vi "Dresden R2R Sputter 03.02.2018 IY24.vi"() -> ()   [LabVIEW 2009] (continued)
                                }
                                frame #1 {
                                }
                                }
                                }
                                frame #1 {
                                }
                                }
                                }
                                frame #5 {
                                n21432 = local read "Semi"() -> (w22479:bool)
                                n21433 = case shown="False" w22479 {
                                frame #0 {
                                n21434 = while {
                                i -> [w22485]
                                stop <- w22481 stop-if-true
                                n21435 = local read "Pc_bv_opened_ch4"() -> (w22483:bool)
                                n21436 = Greater?(x=w22485, y=120) -> (0:w22484:bool)
                                n21437 = local read "Semi"() -> (w22482:bool)
                                n21438 = Compound Arithmetic op=OR(w22482, w22483, w22484) -> (w22481:bool)
                                n21439 = Wait (ms)(milliseconds to wait=u32 500) -> ()  [unwired: 1 out]
                                }
                                }
                                frame #1 {
                                }
                                }
                                }
                                frame #6 {
                                n21440 = local read "Semi"() -> (w22487:bool)
                                n21441 = case shown="False" w22487 {
                                frame #0 {
                                n21442 = local read "Pc_bv_opened_ch4"() -> (w22488:bool)
                                n21443 = case shown="False" w22488 {
                                frame #0 {
                                n21444 = local write "Error Message"("Start up process  cancelled\nbecause  PC-BV not opened.\nPlease check PC-BV4 connections." ("Error Message")) -> ()
                                n21445 = Wait (ms)(milliseconds to wait=u32 1000) -> ()  [unwired: 1 out]
                                }
                                frame #1 {
                                }
                                }
                                }
                                frame #1 {
                                }
                                }
                                }
                                }
                                }
                                frame #1 {
                                }
                                }
                                }
                                frame #1 {
                                n21446 = local read "Semi"() -> (w22491:bool)
                                n21447 = case shown="False" w22491 {
                                frame #0 {
                                n21448 = local write "Ch4_PV13"(TRUE ("P03")) -> ()
                                n21449 = Wait Until Next ms Multiple(millisecond multiple=u32 1000) -> ()  [unwired: 1 out]
                                }
                                frame #1 {
                                }
                                }
                                }
                                }
                              }
                              frame #1 {
                              }
                            }
                          }
                          frame #9 {
                            # "OPEN/CLOSE TRNS GV-BP"
                            n21450 = local read "Semi"() -> (w22494:bool)
                            n21451 = case shown="False" w22494 {
                              frame #0 {
                                n21452 = stacked-sequence {
                                frame #0 {
                                n21453 = local read "Semi"() -> (w22495:bool)
                                n21454 = case shown="False" w22495 {
                                frame #0 {
                                n21455 = while {
                                i -> [w22504]
                                stop <- w22499 stop-if-true
                                n21456 = Greater?(x=w22504, y=50) -> (0:w22502:bool)
                                n21457 = case shown="True" w22502 {
                                frame #0 {
                                }
                                frame #1 {
                                n21458 = local read "Ch3_pressure"() -> (w22518:dbl)
                                n21459 = Less?(x=w22518, y=1) -> (x < y?=w22517:bool)
                                n21460 = case shown="True" w22517 {
                                frame #0 {
                                n21461 = local write "Error Message"("Start up process  cancelled\nbecause \n Trns GV-BP2 not closed.\nPlease check \nTrns GV-BP2 connections." ("Error Message")) -> ()
                                }
                                frame #1 {
                                n21462 = local write "Error Message"("Start up process  cancelled\nbecause\n  Trns GV-BP2 not opened.\nPlease check \nTrns GV-BP2 connections." ("Error Message")) -> ()
                                }
                                }
                                n21463 = local write "Semi"(TRUE ("Semi")) -> ()
                                }
                                }
                                n21464 = local read "Ch3_pressure"() -> (w22498:dbl)
                                n21465 = Less?(x=w22498, y=1) -> (x < y?=w22496:bool)
                                n21466 = case shown="True" w22496 {
                                tunnel: [w22506 w22512] -> w22501
                                frame #0 {
                                n21467 = local read "Ch4_Trns_gv_bp_di"() -> (w22505:bool)
                                n21468 = case shown="True" w22505 {
                                tunnel: [TRUE FALSE] -> w22506
                                frame #0 {
                                }
                                frame #1 {
                                n21469 = local write "Ch4_Trns_gv_bp_do"(FALSE ("Ch1_Tp_bv_do")) -> ()
                                n21470 = Wait Until Next ms Multiple(millisecond multiple=u32 200) -> ()  [unwired: 1 out]
                                }
                                }
                                }
                                frame #1 {
                                n21471 = local read "Ch4_Trns_gv_bp_di"() -> (w22511:bool)
                                n21472 = case shown="False" w22511 {
                                tunnel: [FALSE TRUE] -> w22512
                                frame #0 {
                                n21473 = local write "Ch4_Trns_gv_bp_do"(TRUE ("Ch1_Tp_bv_do")) -> ()
                                n21474 = Wait Until Next ms Multiple(millisecond multiple=u32 200) -> ()  [unwired: 1 out]
                                }
                                frame #1 {
                                }
                                }
                                }
                                }
                                n21475 = local read "Semi"() -> (w22500:bool)
                                n21476 = Or(x=w22501, y=w22500) -> (x .or. y?=w22499:bool)
                                }
                                }
                                frame #1 {
                                }
                                }
                                }
                                frame #1 {
                                n21477 = local read "Semi"() -> (w22523:bool)
                                n21478 = case shown="False" w22523 {
                                frame #0 {
                                n21479 = local write "Ch4_PV14"(TRUE ("P03")) -> ()
                                n21480 = Wait Until Next ms Multiple(millisecond multiple=u32 1000) -> ()  [unwired: 1 out]
                                }
                                frame #1 {
                                }
                                }
                                }
                                }
                              }
                              frame #1 {
                              }
                            }
                          }
                          frame #10 {
                            # "CHECK CH-PRESSURE"
                            n21481 = local read "Semi"() -> (w22526:bool)
                            n21482 = case shown="False" w22526 {
                              frame #0 {
                                n21483 = stacked-sequence {
                                frame #0 {
                                n21484 = local read "Semi"() -> (w22527:bool)
                                n21485 = case shown="False" w22527 {
                                frame #0 {
                                n21486 = while {
                                i -> [w22536]
                                stop <- w22531 stop-if-true
                                n21487 = Greater?(x=w22536, y=600) -> (0:w22534:bool)
                                n21488 = case shown="True" w22534 {
                                frame #0 {
                                }
                                frame #1 {
                                n21489 = local write "Semi"(TRUE ("Semi")) -> ()
                                n21490 = local write "Error Message"("Start up process was cancelled.\nPlease check chamber \nvacuum connections." ("Error Message")) -> ()
                                }
                                }
                                n21491 = local read "Ch4pressure"() -> (w22530:dbl)
                                n21492 = Less?(x=w22530, y=0.9) -> (x < y?=w22528:bool)
                                n21493 = case shown="False" w22528 {
                                tunnel: [FALSE TRUE] -> w22533
                                frame #0 {
                                n21494 = Wait Until Next ms Multiple(millisecond multiple=u32 500) -> ()  [unwired: 1 out]
                                }
                                frame #1 {
                                }
                                }
                                n21495 = local read "Semi"() -> (w22532:bool)
                                n21496 = Or(x=w22533, y=w22532) -> (x .or. y?=w22531:bool)
                                }
                                }
                                frame #1 {
                                }
                                }
                                }
                                frame #1 {
                                n21497 = local read "Semi"() -> (w22542:bool)
                                n21498 = case shown="False" w22542 {
                                frame #0 {
                                n21499 = local write "Ch4_PV15"(TRUE ("P03")) -> ()
                                n21500 = Wait Until Next ms Multiple(millisecond multiple=u32 1000) -> ()  [unwired: 1 out]
                                }
                                frame #1 {
                                }
                                }
                                }
                                }
                              }
                              frame #1 {
                              }
                            }
                          }
                          frame #11 {
                            # "OPEN BG-BV"
                            n21501 = local read "Semi"() -> (w22545:bool)
                            n21502 = case shown="False" w22545 {
                              frame #0 {
                                n21503 = stacked-sequence {
                                frame #0 {
                                n21504 = local read "Semi"() -> (w22546:bool)
                                n21505 = case shown="False" w22546 {
                                frame #0 {
                                n21506 = while {
                                i -> [w22553]
                                stop <- w22548 stop-if-true
                                n21507 = Greater?(x=w22553, y=50) -> (0:w22551:bool)
                                n21508 = case shown="True" w22551 {
                                frame #0 {
                                }
                                frame #1 {
                                n21509 = local write "Semi"(TRUE ("Semi")) -> ()
                                n21510 = local write "Error Message"("Start up process  cancelled\nbecause  BG-BV not opened.\nPlease check BG-BV4 connections." ("Error Message")) -> ()
                                }
                                }
                                n21511 = local read "Ch4_Bg_bv_di"() -> (w22547:bool)
                                n21512 = case shown="False" w22547 {
                                tunnel: [FALSE TRUE] -> w22550
                                frame #0 {
                                n21513 = Wait Until Next ms Multiple(millisecond multiple=u32 200) -> ()  [unwired: 1 out]
                                n21514 = local write "Ch4_Bg_bv_do"(TRUE ("Ch1_Tp_bv_do")) -> ()
                                }
                                frame #1 {
                                }
                                }
                                n21515 = local read "Semi"() -> (w22549:bool)
                                n21516 = Or(x=w22550, y=w22549) -> (x .or. y?=w22548:bool)
                                }
                                }
                                frame #1 {
                                }
                                }
                                }
                                frame #1 {
                                n21517 = local read "Semi"() -> (w22560:bool)
                                n21518 = case shown="False" w22560 {
                                frame #0 {
                                n21519 = local write "Ch4_PV16"(TRUE ("P03")) -> ()
                                n21520 = Wait Until Next ms Multiple(millisecond multiple=u32 1000) -> ()  [unwired: 1 out]
                                }
                                frame #1 {
                                }
                                }
                                }
                                }
                              }
                              frame #1 {
                              }
                            }
                          }
                          frame #12 {
                            # "CHECK CH-PRESSURE"
                            n21521 = local read "Semi"() -> (w22563:bool)
                            n21522 = case shown="False" w22563 {
                              frame #0 {
                                n21523 = stacked-sequence {
                                frame #0 {
                                n21524 = local read "Semi"() -> (w22564:bool)
                                n21525 = case shown="False" w22564 {
                                frame #0 {
                                n21526 = while {
                                i -> [w22573]
                                stop <- w22568 stop-if-true
                                n21527 = Greater?(x=w22573, y=240) -> (0:w22571:bool)
                                n21528 = case shown="True" w22571 {
                                frame #0 {
                                }
                                frame #1 {
                                n21529 = local write "Semi"(TRUE ("Semi")) -> ()
                                n21530 = local write "Error Message"("Start up process was cancelled.\nPlease check chamber \nvacuum connections." ("Error Message")) -> ()
                                }
                                }
                                n21531 = local read "Ch4pressure"() -> (w22567:dbl)
                                n21532 = Less?(x=w22567, y=0.9) -> (x < y?=w22565:bool)
                                n21533 = case shown="False" w22565 {
                                tunnel: [FALSE TRUE] -> w22570
                                frame #0 {
                                n21534 = Wait Until Next ms Multiple(millisecond multiple=u32 500) -> ()  [unwired: 1 out]
                                }
                                frame #1 {
                                }
                                }
                                n21535 = local read "Semi"() -> (w22569:bool)
                                n21536 = Or(x=w22570, y=w22569) -> (x .or. y?=w22568:bool)
                                }
                                }
                                frame #1 {
                                }
                                }
                                }
                                frame #1 {
                                n21537 = local read "Semi"() -> (w22579:bool)
                                n21538 = case shown="False" w22579 {
                                frame #0 {
                                n21539 = local write "Ch4_PV17"(TRUE ("P03")) -> ()
                                n21540 = Wait Until Next ms Multiple(millisecond multiple=u32 1000) -> ()  [unwired: 1 out]
                                }
                                frame #1 {
                                }
                                }
                                }
                                }
                              }
                              frame #1 {
                              }
                            }
                          }
                          frame #13 {
                            # "START TP"
                            n21541 = local read "Semi"() -> (w22582:bool)
                            n21542 = case shown="False" w22582 {
                              frame #0 {
                                n21543 = stacked-sequence {
                                frame #0 {
                                n21544 = local read "Semi"() -> (w22583:bool)
                                n21545 = case shown="False" w22583 {
                                frame #0 {
                                n21546 = stacked-sequence {
                                frame #0 {
                                n21547 = local read "Semi"() -> (w22584:bool)
                                n21548 = case shown="False" w22584 {
                                frame #0 {
                                n21549 = local write "Tp4_auto_start"(TRUE ("Tp1_auto_start")) -> ()
                                }
                                frame #1 {
                                }
                                }
                                }
                                frame #1 {
                                n21550 = local read "Semi"() -> (w22586:bool)
                                n21551 = case shown="False" w22586 {
                                frame #0 {
                                n21552 = Wait (ms)(milliseconds to wait=u32 1000) -> ()  [unwired: 1 out]
                                }
                                frame #1 {
                                }
                                }
                                }
                                frame #2 {
                                n21553 = local read "Semi"() -> (w22588:bool)
                                n21554 = case shown="False" w22588 {
                                frame #0 {
                                n21555 = while {
                                i -> [w22594]
                                stop <- w22590 stop-if-true
                                n21556 = local read "TP4_working"() -> (w22592:bool)
                                n21557 = Greater?(x=w22594, y=120) -> (0:w22593:bool)
                                n21558 = local read "Semi"() -> (w22591:bool)
                                n21559 = Compound Arithmetic op=OR(w22591, w22592, w22593) -> (w22590:bool)
                                n21560 = Wait (ms)(milliseconds to wait=u32 500) -> ()  [unwired: 1 out]
                                }
                                }
                                frame #1 {
                                }
                                }
                                }
                                frame #3 {
                                n21561 = local read "Semi"() -> (w22596:bool)
                                n21562 = case shown="False" w22596 {
                                frame #0 {
                                n21563 = local read "TP4_working"() -> (w22597:bool)
                                n21564 = case shown="False" w22597 {
                                frame #0 {
                                n21565 = local write "Tp4_auto_start"(TRUE ("Pc_bv1_auto_open")) -> ()
                                }
                                frame #1 {
                                }
                                }
                                }
                                frame #1 {
                                }
                                }
                                }
                                frame #4 {
                                n21566 = local read "Semi"() -> (w22599:bool)
                                n21567 = case shown="False" w22599 {
                                frame #0 {
                                n21568 = local read "TP4_working"() -> (w22600:bool)
                                n21569 = case shown="False" w22600 {
                                frame #0 {
                                n21570 = Wait (ms)(milliseconds to wait=u32 1000) -> ()  [unwired: 1 out]
                                }
                                frame #1 {
                                }
                                }
                                }
                                frame #1 {
                                }
                                }
                                }
                                frame #5 {
                                n21571 = local read "Semi"() -> (w22602:bool)
                                n21572 = case shown="False" w22602 {
                                frame #0 {
                                n21573 = while {
                                i -> [w22608]
                                stop <- w22604 stop-if-true
                                n21574 = local read "TP4_working"() -> (w22606:bool)
                                n21575 = Greater?(x=w22608, y=120) -> (0:w22607:bool)
                                n21576 = local read "Semi"() -> (w22605:bool)
                                n21577 = Compound Arithmetic op=OR(w22605, w22606, w22607) -> (w22604:bool)
                                n21578 = Wait (ms)(milliseconds to wait=u32 500) -> ()  [unwired: 1 out]
                                }
                                }
                                frame #1 {
                                }
                                }
                                }
                                frame #6 {
                                n21579 = local read "Semi"() -> (w22610:bool)
                                n21580 = case shown="False" w22610 {
                                frame #0 {
                                n21581 = local read "TP4_working"() -> (w22611:bool)
                                n21582 = case shown="False" w22611 {
                                frame #0 {
                                n21583 = local write "Error Message"("Start up process  cancelled\nbecause  TP not started.\nPlease check TP4 connections." ("Error Message")) -> ()
                                n21584 = Wait (ms)(milliseconds to wait=u32 1000) -> ()  [unwired: 1 out]
                                }
                                frame #1 {
                                }
                                }
                                }
                                frame #1 {
                                }
                                }
                                }
                                }
                                }
                                frame #1 {
                                }
                                }
                                }
                                frame #1 {
                                n21585 = local read "Semi"() -> (w22614:bool)
                                n21586 = case shown="False" w22614 {
                                frame #0 {
                                n21587 = Wait Until Next ms Multiple(millisecond multiple=u32 1000) -> ()  [unwired: 1 out]
                                n21588 = local write "Ch4_PV18"(TRUE ("P03")) -> ()
                                }
                                frame #1 {
                                }
                                }
                                }
                                }
                              }
                              frame #1 {
                              }
                            }
                          }
                        }
                      }
                      frame #1 {
                      }
                    }
                  }
                  frame #1 {
                    # "PUMPING CH3 HIGHER THAN 0.9 TORR"
                    n21589 = local read "Semi"() -> (w22617:bool)
                    n21590 = case shown="False" w22617 {
                      frame #0 {
                        n21591 = stacked-sequence {
                          frame #0 {
                            # "STOP TP"
                            n21592 = local read "Semi"() -> (w22618:bool)
                            n21593 = case shown="False" w22618 {
                              frame #0 {
                                n21594 = stacked-sequence {
                                frame #0 {
                                n21595 = local read "Semi"() -> (w22619:bool)
                                n21596 = case shown="False" w22619 {
                                frame #0 {
                                n21597 = stacked-sequence {
                                frame #0 {
                                n21598 = local read "Semi"() -> (w22620:bool)
                                n21599 = case shown="False" w22620 {
                                frame #0 {
                                n21600 = local write "Tp4_auto_stop"(TRUE ("Tp1_auto_start")) -> ()
                                }
                                frame #1 {
                                }
                                }
                                }
                                frame #1 {
                                n21601 = local read "Semi"() -> (w22622:bool)
                                n21602 = case shown="False" w22622 {
                                frame #0 {
                                n21603 = Wait (ms)(milliseconds to wait=u32 1000) -> ()  [unwired: 1 out]
                                }
                                frame #1 {
                                }
                                }
                                }
                                frame #2 {
                                n21604 = local read "Semi"() -> (w22624:bool)
                                n21605 = case shown="False" w22624 {
                                frame #0 {
                                n21606 = while {
                                i -> [w22630]
                                stop <- w22626 stop-if-true
                                n21607 = local read "Tp4_stopped"() -> (w22628:bool)
                                n21608 = Greater?(x=w22630, y=120) -> (0:w22629:bool)
                                n21609 = local read "Semi"() -> (w22627:bool)
                                n21610 = Compound Arithmetic op=OR(w22627, w22628, w22629) -> (w22626:bool)
                                n21611 = Wait (ms)(milliseconds to wait=u32 500) -> ()  [unwired: 1 out]
                                }
                                }
                                frame #1 {
                                }
                                }
                                }
                                frame #3 {
                                n21612 = local read "Semi"() -> (w22632:bool)
                                n21613 = case shown="False" w22632 {
                                frame #0 {
                                n21614 = local read "Tp4_stopped"() -> (w22633:bool)
                                n21615 = case shown="False" w22633 {
                                frame #0 {
                                n21616 = local write "Tp4_auto_stop"(TRUE ("Pc_bv1_auto_open")) -> ()
                                }
                                frame #1 {
                                }
                                }
                                }
                                frame #1 {
                                }
                                }
                                }
                                frame #4 {
                                n21617 = local read "Semi"() -> (w22635:bool)
                                n21618 = case shown="False" w22635 {
                                frame #0 {
                                n21619 = local read "Tp4_stopped"() -> (w22636:bool)
                                n21620 = case shown="False" w22636 {
                                frame #0 {
                                n21621 = Wait (ms)(milliseconds to wait=u32 1000) -> ()  [unwired: 1 out]
                                }
                                frame #1 {
                                }
                                }
                                }
                                frame #1 {
                                }
                                }
                                }
                                frame #5 {
                                n21622 = local read "Semi"() -> (w22638:bool)
                                n21623 = case shown="False" w22638 {
                                frame #0 {
                                n21624 = while {
                                i -> [w22644]
                                stop <- w22640 stop-if-true
                                n21625 = local read "Tp4_stopped"() -> (w22642:bool)
                                n21626 = Greater?(x=w22644, y=120) -> (0:w22643:bool)
                                n21627 = local read "Semi"() -> (w22641:bool)
                                n21628 = Compound Arithmetic op=OR(w22641, w22642, w22643) -> (w22640:bool)
                                n21629 = Wait (ms)(milliseconds to wait=u32 500) -> ()  [unwired: 1 out]
                                }
                                }
                                frame #1 {
                                }
                                }
                                }
                                frame #6 {
                                n21630 = local read "Semi"() -> (w22646:bool)
                                n21631 = case shown="False" w22646 {
                                frame #0 {
                                n21632 = local read "Tp4_stopped"() -> (w22647:bool)
                                n21633 = case shown="False" w22647 {
                                frame #0 {
                                n21634 = local write "Error Message"("Start up process  cancelled\nbecause  TP not stopped.\nPlease check TP4 connections." ("Error Message")) -> ()
                                n21635 = Wait (ms)(milliseconds to wait=u32 1000) -> ()  [unwired: 1 out]
                                }
                                frame #1 {
                                }
                                }
                                }
                                frame #1 {
                                }
                                }
                                }
                                }
                                }
                                frame #1 {
                                }
                                }
                                }
                                frame #1 {
                                n21636 = local read "Semi"() -> (w22650:bool)
                                n21637 = case shown="False" w22650 {
                                frame #0 {
                                n21638 = local write "Ch4_PA5"(TRUE ("PA2")) -> ()
                                n21639 = Wait Until Next ms Multiple(millisecond multiple=u32 1000) -> ()  [unwired: 1 out]
                                }
                                frame #1 {
                                }
                                }
                                }
                                }
                              }
                              frame #1 {
                              }
                            }
                          }
                          frame #1 {
                            # "CLOSE CH1-CC"
                            n21640 = local read "Semi"() -> (w22653:bool)
                            n21641 = case shown="False" w22653 {
                              frame #0 {
                                n21642 = stacked-sequence {
                                frame #0 {
                                n21643 = local read "Semi"() -> (w22654:bool)
                                n21644 = case shown="False" w22654 {
                                frame #0 {
                                n21645 = while {
                                i -> [w22661]
                                stop <- w22655 stop-if-true
                                n21646 = Greater?(x=w22661, y=50) -> (0:w22659:bool)
                                n21647 = case shown="True" w22659 {
                                frame #0 {
                                }
                                frame #1 {
                                n21648 = local write "Semi"(TRUE ("Semi")) -> ()
                                n21649 = local write "Error Message"("Start up process  cancelled\nbecause  CH-CC not closed.\nPlease check  CH4-CC connections." ("Error Message")) -> ()
                                }
                                }
                                n21650 = local read "Ch4_Cc_on_off_di"() -> (w22658:bool)
                                n21651 = case shown="True" w22658 {
                                tunnel: [TRUE FALSE] -> w22657
                                frame #0 {
                                }
                                frame #1 {
                                n21652 = Wait Until Next ms Multiple(millisecond multiple=u32 200) -> ()  [unwired: 1 out]
                                n21653 = local write "Ch4_Cc_on_off_do"(FALSE ("Ch1_Tp_bv_do")) -> ()
                                }
                                }
                                n21654 = local read "Semi"() -> (w22656:bool)
                                n21655 = Or(x=w22657, y=w22656) -> (x .or. y?=w22655:bool)
                                }
                                }
                                frame #1 {
                                }
                                }
                                }
                                frame #1 {
                                n21656 = local read "Semi"() -> (w22668:bool)
                                n21657 = case shown="False" w22668 {
                                frame #0 {
                                n21658 = local write "Ch4_PA6"(TRUE ("PA3")) -> ()
                                n21659 = Wait Until Next ms Multiple(millisecond multiple=u32 1000) -> ()  [unwired: 1 out]
                                }
                                frame #1 {
                                }
                                }
                                }
                                }
                              }
                              frame #1 {
                              }
                            }
                          }
                          frame #2 {
                            # "CLOSE BG-BV"
                            n21660 = local read "Semi"() -> (w22671:bool)
                            n21661 = case shown="False" w22671 {
                              frame #0 {
                                n21662 = stacked-sequence {
                                frame #0 {
                                n21663 = local read "Semi"() -> (w22672:bool)
                                n21664 = case shown="False" w22672 {
                                frame #0 {
                                n21665 = while {
                                i -> [w22679]
                                stop <- w22673 stop-if-true
                                n21666 = Greater?(x=w22679, y=50) -> (0:w22677:bool)
                                n21667 = case shown="True" w22677 {
                                frame #0 {
                                }
                                frame #1 {
                                n21668 = local write "Semi"(TRUE ("Semi")) -> ()
                                n21669 = local write "Error Message"("Start up process  cancelled\nbecause  BG-BV not closed.\nPlease check  BG-BV4 connections." ("Error Message")) -> ()
                                }
                                }
                                n21670 = local read "Ch4_Bg_bv_di"() -> (w22676:bool)
                                n21671 = case shown="True" w22676 {
                                tunnel: [TRUE FALSE] -> w22675
                                frame #0 {
                                }
                                frame #1 {
                                n21672 = Wait Until Next ms Multiple(millisecond multiple=u32 200) -> ()  [unwired: 1 out]
                                n21673 = local write "Ch4_Bg_bv_do"(FALSE ("Ch1_Tp_bv_do")) -> ()
                                }
                                }
                                n21674 = local read "Semi"() -> (w22674:bool)
                                n21675 = Or(x=w22675, y=w22674) -> (x .or. y?=w22673:bool)
                                }
                                }
                                frame #1 {
                                }
                                }
                                }
                                frame #1 {
                                n21676 = local read "Semi"() -> (w22686:bool)
                                n21677 = case shown="False" w22686 {
                                frame #0 {
                                n21678 = local write "Ch4_PA7"(TRUE ("PA3")) -> ()
                                n21679 = Wait Until Next ms Multiple(millisecond multiple=u32 1000) -> ()  [unwired: 1 out]
                                }
                                frame #1 {
                                }
                                }
                                }
                                }
                              }
                              frame #1 {
                              }
                            }
                          }
                          frame #3 {
                            # "CLOSE TP-BV"
                            n21680 = local read "Semi"() -> (w22689:bool)
                            n21681 = case shown="False" w22689 {
                              frame #0 {
                                n21682 = stacked-sequence {
                                frame #0 {
                                n21683 = local read "Semi"() -> (w22690:bool)
                                n21684 = case shown="False" w22690 {
                                frame #0 {
                                n21685 = while {
                                i -> [w22697]
                                stop <- w22691 stop-if-true
                                n21686 = Greater?(x=w22697, y=50) -> (0:w22695:bool)
                                n21687 = case shown="True" w22695 {
                                frame #0 {
                                }
                                frame #1 {
                                n21688 = local write "Semi"(TRUE ("Semi")) -> ()
                                n21689 = local write "Error Message"("Start up process  cancelled\nbecause  TP-BV not closed.\nPlease check  TP4-BV connections." ("Error Message")) -> ()
                                }
                                }
                                n21690 = local read "Ch4_Tp_bv_di"() -> (w22694:bool)
                                n21691 = case shown="True" w22694 {
                                tunnel: [TRUE FALSE] -> w22693
                                frame #0 {
                                }
                                frame #1 {
                                n21692 = Wait Until Next ms Multiple(millisecond multiple=u32 200) -> ()  [unwired: 1 out]
                                n21693 = local write "Ch4_Tp_bv_do"(FALSE ("Ch1_Tp_bv_do")) -> ()
                                }
                                }
                                n21694 = local read "Semi"() -> (w22692:bool)
                                n21695 = Or(x=w22693, y=w22692) -> (x .or. y?=w22691:bool)
                                }
                                }
                                frame #1 {
                                }
                                }
                                }
                                frame #1 {
                                n21696 = local read "Semi"() -> (w22704:bool)
                                n21697 = case shown="False" w22704 {
                                frame #0 {
                                n21698 = local write "Ch4_PA8"(TRUE ("PA5")) -> ()
                                n21699 = Wait Until Next ms Multiple(millisecond multiple=u32 1000) -> ()  [unwired: 1 out]
                                }
                                frame #1 {
                                }
                                }
                                }
                                }
                              }
                              frame #1 {
                              }
                            }
                          }
                          frame #4 {
                            # "False PL1-ATM"
                            n21700 = local read "Semi"() -> (w22707:bool)
                            n21701 = case shown="False" w22707 {
                              frame #0 {
                                n21702 = stacked-sequence {
                                frame #0 {
                                n21703 = local read "Semi"() -> (w22708:bool)
                                n21704 = case shown="False" w22708 {
                                frame #0 {
                                n21705 = local write "Ch4_Pl_atm_do"(FALSE ("Ch1_Pl_atm_do")) -> ()
                                }
                                frame #1 {
                                }
                                }
                                }
                                frame #1 {
                                n21706 = local read "Semi"() -> (w22710:bool)
                                n21707 = case shown="False" w22710 {
                                frame #0 {
                                n21708 = local write "Ch4_PA9"(TRUE ("PA3")) -> ()
                                n21709 = Wait Until Next ms Multiple(millisecond multiple=u32 1000) -> ()  [unwired: 1 out]
                                }
                                frame #1 {
                                }
                                }
                                }
                                }
                              }
                              frame #1 {
                              }
                            }
                          }
                          frame #5 {
                            # "STOP MP"
                            n21710 = local read "Semi"() -> (w22713:bool)
                            n21711 = case shown="False" w22713 {
                              frame #0 {
                                n21712 = stacked-sequence {
                                frame #0 {
                                n21713 = local read "Semi"() -> (w22714:bool)
                                n21714 = case shown="False" w22714 {
                                frame #0 {
                                n21715 = while {
                                i -> [w22721]